vi "UHR-Fleezers Control (host) - Avogadro v3.vi"() -> ()   [LabVIEW 2014] (continued)
  n68 = Bundle("New Image"=w50, "New Image"=w49, "New Image"=w32, "New Image"=w48, "New Image"=w47) -> (w46:T42)  [unwired: 1 in]
  n69 = call-poly "VISA Configure Serial Port"("VISA resource name"=refnum<visa-resource-name> "COM5", "timeout (10sec)"=u32 1000, "baud rate (9600)"=u32 19200) -> ("VISA resource name out"=w3:refnum<visa-resource-name>, "error out"=w6:errorcluster)  [unwired: 4 in, 7 out]
  "Stage Control Serial Error" <- w6
  n70 = node-c288() -> (w53:T43)  [unwired: 4 in]
  n71 = timed-loop "Run Scripts, including: stage motion" {
    tunnel: w6 -> [w231]
    tunnel: w3 -> [w232]
    tunnel: [w232] -> w55
    tunnel: [w231] -> w54
    timing: w53 -> [_]
    timing-out: [_] -> w52
    tunnel: w44 -> [w230]
    tunnel: w45 -> [w229]
    tunnel: w40 -> [w226]
    tunnel: w39 -> [w225]
    tunnel: w38 -> [w227]
    tunnel: w37 -> [w228]
    tunnel: w29 -> [w224]
    tunnel: w26 -> [w223]
    tunnel: w14 -> [w222]
    tunnel: w13 -> [w221]
    stop <- w233 stop-if-true
    n72 = node-c288() -> ()  [unwired: 1 in, 1 out]
    n73 = event shown="[13] \"Cal/Data Acq. Spot\": Value Change" {
      selector: _ -> [_ _ _ _ _ _ _ _ _ _ _ _ _ _ _ _ _ _ _ _ _ _ _ _ _ _ _]
      dyn-events: _ -> [_ _ _ _ _ _ _ _ _ _ _ _ _ _ _ _ _ _ _ _ _ _ _ _ _ _ _]
      timeout: _ -> [_ _ _ _ _ _ _ _ _ _ _ _ _ _ _ _ _ _ _ _ _ _ _ _ _ _ _]
      tunnel: ["Set Position" _ "Move to Position" _ _ _ _ _ _ "Read Harvard" _ _ _ _ _ _ _ _ "Force FB Data\nScript" _ _ "Take Stepping Data" _ "Take Detection Laser\nImage" _ _ _] -> _
      tunnel: [_ _ _ _ _ _ _ _ _ _ _ _ _ _ _ _ _ _ _ _ _ _ _ _ _ w1240 _] -> w233
      tunnel: w231 -> [w252 w260 w271 w284 w314 _ _ _ _ _ w451 w485 w511 w544 w653 w682 w814 w842 w873 _ _ _ _ _ _ _ _]
      tunnel: w232 -> [w253 w261 w272 w285 w315 _ _ _ _ _ w452 w486 w512 w545 w654 w683 w815 w843 w874 _ _ _ _ _ _ _ _]
      tunnel: w230 -> [_ _ _ _ _ _ _ _ _ w436 _ _ _ _ _ _ _ _ _ _ _ _ _ _ _ _ _]
      tunnel: w229 -> [_ _ _ _ _ _ _ _ _ w435 _ _ _ _ _ _ _ _ _ _ _ _ _ _ _ _ _]
      tunnel: w228 -> [_ _ _ _ _ _ _ _ _ _ _ _ _ _ _ _ _ _ _ _ _ _ _ _ _ _ _]
      tunnel: w227 -> [_ _ _ _ _ _ _ _ _ _ _ _ _ _ _ _ _ _ _ _ _ _ _ _ _ _ _]
      tunnel: w226 -> [_ _ _ _ _ _ _ _ _ _ _ _ _ _ _ _ _ _ _ _ _ _ _ _ _ _ _]
      tunnel: w225 -> [_ _ _ _ _ _ _ _ _ _ _ _ _ _ _ _ _ _ _ _ _ _ _ _ _ _ _]
      tunnel: w224 -> [_ _ _ _ _ w342 w349 w377 w396 _ _ _ _ _ _ _ _ _ _ _ _ _ _ _ _ w1239 _]
      tunnel: w223 -> [_ _ _ _ _ _ _ _ _ _ _ _ _ w537 _ _ _ _ _ _ _ _ _ _ w1106 _ _]
      tunnel: w222 -> [_ _ _ _ _ _ _ _ _ _ _ _ _ _ _ _ _ _ _ _ _ _ _ _ _ _ w1250]
      tunnel: w221 -> [_ _ _ _ _ _ _ _ _ _ _ _ _ _ _ _ _ _ _ _ _ _ _ _ _ _ w1245]
      event "Set Position", "Set Position 2", "Set Position 3", "Set Position 4", "Set Position 5", "Set Position 1", "Set Position 6": Value Change {
        n74 = event-data() -> ()  [unwired: 1 in, 5 out]
        n75 = Build Array("Set Position 1", "Set Position 2", "Set Position 3", "Set Position 4", "Set Position 5", "Set Position 6") -> (w251:bool[])
        n76 = Boolean Array To Number(Boolean array=w251) -> (number=w250:u32)
        n77 = Logarithm Base 2(1:w250) -> (0:w242:dbl)
        n78 = call "Read Stage Position.vi"("error in"=w252, "VISA resource name in"=w253) -> ("Current Position"=w257:cluster{dbl, dbl, dbl}, "error out"=w256:errorcluster)  [unwired: 2 out]
        n79 = Decrement(x="Position") -> (x-1=w240:dbl)
        n80 = Greater Or Equal?(x=w242, y=0.0) -> (x >= y?=w243:bool)
        n81 = Cluster To Array(cluster=w257) -> (array=w254:dbl[])
        n82 = Select(t=w242, s=w243, f=w240) -> (s? t:f=w239:dbl)
        n83 = local write "Stage Control Serial Error"(w256) -> ()
        n84 = Increment(x=w239) -> (x+1=w238:dbl)
        n85 = Build Array (concatenate)(w238, w254) -> (w237:dbl[])
        n86 = Replace Array Subset(array="Saved Stage Positions", new element=w237, index (row)=w239) -> (w255:dbl[][])  [unwired: 1 in]
        n87 = local write "Saved Stage Positions"(w255) -> ()
      }
      event Menu Selection (User) {
        n88 = event-data() -> ("ItemTag"=w262:string)  [unwired: 1 in, 6 out]
        n89 = case shown="\"Z\"" w262 {
          tunnel: w261 -> [_ w264 w269 _]
          tunnel: w260 -> [_ w263 w267 _]
          frame "False", Default {
          }
          frame "XY" {
            n90 = call "start_stage_trackball.vi"("Enum"=T46."Trackball XY", "error in (no error)"=w263, "Stage Controller port"=w264) -> ("error out"=w266:errorcluster)  [unwired: 1 out]
            n91 = property on="Stage Control Serial Error" class="Clust (strict)"("Val(Sgnl)"=w266) -> ()  [unwired: 2 in, 2 out]
          }
          frame "Z" {
            n92 = call "start_stage_trackball.vi"("Enum"=T46."Trackball Z", "error in (no error)"=w267, "Stage Controller port"=w269) -> ("error out"=w268:errorcluster)  [unwired: 1 out]
            n93 = property on="Stage Control Serial Error" class="Clust (strict)"("Val(Sgnl)"=w268) -> ()  [unwired: 2 in, 2 out]
          }
          frame "True" {
          }
        }
      }
      event "Move to Position": Value Change {
        n94 = event-data() -> ()  [unwired: 1 in, 5 out]
        n95 = flat-sequence {
          tunnel: w272 -> [w276]
          tunnel: w271 -> [w275]
          frame #0 {
            n96 = local read "Saved Stage Positions"() -> (w278:dbl[][])
            n97 = local read "Position"() -> (w277:dbl)
            n98 = local write "Stage Moving"(TRUE ("Stage Moving")) -> ()
            n99 = call "move to saved stage position.vi"("error in"=w275, "Stage VISA resource name in"=w276, "Position"=w277, "Saved Stage Positions"=w278) -> ("error out"=w274:errorcluster)  [unwired: 1 out]
            n100 = local write "Stage Control Serial Error"(w274) -> ()
          }
          frame #1 {
            n101 = call <vilib>:"Beep.vi"() -> ()  [unwired: 3 in, 9 out]
            n102 = local write "Stage Moving"(FALSE ("Stage Moving")) -> ()
          }
        }
      }
      event "Move Cap. 1 (DNA Bottom)": Value Change {
        n103 = event-data() -> ()  [unwired: 1 in, 5 out]
        n104 = local write "Move Cap. 1 (DNA Bottom)"(FALSE ("Move Cap. 1 (DNA Right)")) -> ()
        n105 = flat-sequence {
          tunnel: w284 -> [w287]
          tunnel: w285 -> [w288]
          tunnel: [w288] -> w282
          tunnel: [w287] -> w281
          tunnel: w282 -> [w290]
          tunnel: w281 -> [w289]
          frame #0 {
            n106 = property on="Sample Channel\nFlow" class="Bool (strict)"("Val(Sgnl)"="Cap 1 Samp Flow ON") -> ()  [unwired: 2 in, 2 out]
          }
          frame #1 {
            n107 = local read "Saved Stage Positions"() -> (w300:dbl[][])
            n108 = local write "Stage Moving"(TRUE ("Stage Moving")) -> ()
            n109 = Array Subset(array=w300, index (row)=0 ("index"), length (row)=1 ("length"), index (col)=1 ("index"), length (col)=3 ("length")) -> (w297:dbl[][])
            n110 = Reshape Array(w297, 3 ("dimension size")) -> (w295:dbl[])
            n111 = Array To Cluster(array=w295) -> (cluster=w294:cluster{"[0]":dbl, "[1]":dbl, "[2]":dbl})
            n112 = call "Set Stage Position.vi"("Position"=w294, "error in"=w289, "VISA resource name in"=w290) -> ("error out"=w293:errorcluster)  [unwired: 2 out]
            n113 = local write "Stage Control Serial Error"(w293) -> ()
          }
          frame #2 {
            n114 = local write "Stage Moving"(FALSE ("Stage Moving")) -> ()
            n115 = case shown="True" "Cap 1 Flow ON" {
              frame False {
              }
              frame True {
                n116 = property on="Inject Pump 1" class="Bool (strict)"("Val(Sgnl)"=TRUE ("Value (Signaling)")) -> ()  [unwired: 2 in, 2 out]
              }
            }
            n117 = call <vilib>:"Beep.vi"() -> ()  [unwired: 3 in, 9 out]
          }
          frame #3 {
            n118 = property on="Sample Channel\nFlow" class="Bool (strict)"("Val(Sgnl)"=FALSE ("Value (Signaling)")) -> ()  [unwired: 2 in, 2 out]
            n119 = local read "Cap. 2 BD T1?\n(ADig T1, DNA T2)"() -> (w307:bool)
            n120 = case shown="True" w307 {
              tunnel: "Cap 1 T ON" -> [w309 w310]
              frame False {
                n121 = property on="Trap 1 (ON/OFF)" class="Bool (strict)"("Val(Sgnl)"=w309) -> ()  [unwired: 2 in, 2 out]
              }
              frame True {
                n122 = property on="Trap 2 (ON/OFF)" class="Bool (strict)"("Val(Sgnl)"=w310) -> ()  [unwired: 2 in, 2 out]
              }
            }
            n123 = property on="Get bead 2" class="Bool (strict)"("Key Focus"=TRUE) -> ()  [unwired: 2 in, 2 out]
          }
        }
      }
      event "Move Cap. 2 (ADig Top)": Value Change {
        n124 = event-data() -> ()  [unwired: 1 in, 5 out]
        n125 = local write "Move Cap. 2 (ADig Top)"(FALSE ("Move Cap. 2 (ADig Left)")) -> ()
        n126 = flat-sequence {
          tunnel: w314 -> [w317]
          tunnel: w315 -> [w318]
          tunnel: [w318] -> w312
          tunnel: [w317] -> w311
          tunnel: w312 -> [w321]
          tunnel: w311 -> [w320]
          frame #0 {
            n127 = property on="Sample Channel\nFlow" class="Bool (strict)"("Val(Sgnl)"="Cap 2 Samp Flow ON") -> ()  [unwired: 2 in, 2 out]
          }
          frame #1 {
            w319 = FALSE ("Value (Signaling)")
            n128 = local read "Saved Stage Positions"() -> (w331:dbl[][])
            n129 = local write "Stage Moving"(TRUE ("Stage Moving")) -> ()
            n130 = Array Subset(array=w331, index (row)=1 ("index"), length (row)=1 ("length"), index (col)=1 ("index"), length (col)=3 ("length")) -> (w328:dbl[][])
            n131 = Reshape Array(w328, 3 ("dimension size")) -> (w326:dbl[])
            n132 = property on="Trap 1 (ON/OFF)" class="Bool (strict)"("Val(Sgnl)"=w319) -> ()  [unwired: 2 in, 2 out]
            n133 = property on="Trap 1 (ON/OFF)" class="Bool (strict)"("Val(Sgnl)"=w319) -> ()  [unwired: 2 in, 2 out]
            n134 = Array To Cluster(array=w326) -> (cluster=w325:cluster{"[0]":dbl, "[1]":dbl, "[2]":dbl})
            n135 = call "Set Stage Position.vi"("Position"=w325, "error in"=w320, "VISA resource name in"=w321) -> ("error out"=w324:errorcluster)  [unwired: 2 out]
            n136 = local write "Stage Control Serial Error"(w324) -> ()
          }
          frame #2 {
            n137 = local write "Stage Moving"(FALSE ("Stage Moving")) -> ()
            n138 = call <vilib>:"Beep.vi"() -> ()  [unwired: 3 in, 9 out]
            n139 = case shown="True" "Cap 2 Flow ON" {
              frame False {
              }
              frame True {
                n140 = property on="Inject Pump 3" class="Bool (strict)"("Val(Sgnl)"=TRUE ("Value (Signaling)")) -> ()  [unwired: 2 in, 2 out]
              }
            }
          }
          frame #3 {
            n141 = property on="Sample Channel\nFlow" class="Bool (strict)"("Val(Sgnl)"=FALSE ("Value (Signaling)")) -> ()  [unwired: 2 in, 2 out]
            n142 = case shown="False" "Cap. 2 BD T1?\n(ADig T1, DNA T2)" {
              tunnel: "Cap 2 T ON" -> [w340 w341]
              frame False {
                n143 = property on="Trap 2 (ON/OFF)" class="Bool (strict)"("Val(Sgnl)"=w340) -> ()  [unwired: 2 in, 2 out]
              }
              frame True {
                n144 = property on="Trap 1 (ON/OFF)" class="Bool (strict)"("Val(Sgnl)"=w341) -> ()  [unwired: 2 in, 2 out]
              }
            }
            n145 = property on="Get bead 3" class="Bool (strict)"("Key Focus"=TRUE) -> ()  [unwired: 2 in, 2 out]
          }
        }
      }
      event "Send string\nto Blue Laser": Value Change {
        n146 = event-data() -> ()  [unwired: 1 in, 5 out]
        n147 = flat-sequence {
          tunnel: w342 -> [w343]
          frame #0 {
            n148 = call "serial write macro.vi"("String"="command string", "Delay (ms)"="Delay (ms)", "VISA resource name"=w343) -> ("read buffer"=→"read blue buffer":string, "error out"=→"Blue Error Out":errorcluster)  [unwired: 1 out]
            "command string sent" <- "command string"
          }
          frame #1 {
            n149 = local write "Send string\nto Blue Laser"(FALSE ("Send string")) -> ()
          }
        }
      }
      event "Get Blue Laser State": Value Change {
        n150 = event-data() -> ()  [unwired: 1 in, 5 out]
        n151 = local read "Delay (ms)"() -> (w350:i32)
        n152 = flat-sequence {
          tunnel: w350 -> [w358]
          tunnel: w349 -> [w361]
          tunnel: [w359] -> w354
          tunnel: [w358] -> w353
          tunnel: [w368] -> w352
          tunnel: [w365] -> w351
          tunnel: w354 -> [w366]
          tunnel: w353 -> [w365]
          tunnel: w352 -> [w374]
          tunnel: w351 -> [w372]
          frame #0 {
            w356 = "l?"
            n153 = local write "command string sent"(w356) -> ()
            n154 = call "serial write macro.vi"("String"=w356, "Delay (ms)"=w358, "VISA resource name"=w361) -> ("read buffer"=w357:string, "VISA resource name out"=w359:refnum<visa-resource-name>)  [unwired: 1 out]
            n155 = Decimal String To Number(string=w357) -> (number=w360:i32)  [unwired: 2 in, 1 out]
            n156 = Not Equal To 0?(x=w360) -> (x != 0?=→"Laser On":bool)
            n157 = local write "read blue buffer"(w357) -> ()
          }
          frame #1 {
            w363 = "games?" ("String")
            n158 = local write "command string sent"(w363) -> ()
            n159 = call "serial write macro.vi"("String"=w363, "Delay (ms)"=w365, "VISA resource name"=w366) -> ("read buffer"=w364:string, "VISA resource name out"=w368:refnum<visa-resource-name>)  [unwired: 1 out]
            n160 = Decimal String To Number(string=w364) -> (number=w367:i32)  [unwired: 2 in, 1 out]
            n161 = local write "read blue buffer"(w364) -> ()
            n162 = Not Equal To 0?(x=w367) -> (x != 0?=→"Analog Modulation":bool)
          }
          frame #2 {
            w370 = "gdmes?" ("String")
            n163 = local write "command string sent"(w370) -> ()
            n164 = call "serial write macro.vi"("String"=w370, "Delay (ms)"=w372, "VISA resource name"=w374) -> ("read buffer"=w371:string)  [unwired: 2 out]
            n165 = Decimal String To Number(string=w371) -> (number=w373:i32)  [unwired: 2 in, 1 out]
            n166 = Not Equal To 0?(x=w373) -> (x != 0?=→"Digital Modulation":bool)
            n167 = local write "read blue buffer"(w371) -> ()
          }
          frame #3 {
            n168 = local write "Get Blue Laser State"(FALSE) -> ()
          }
        }
      }
      event "Blue Laser Power (mW)\n(Constant Power Mode)", "Blue Laser Modulation\nPower (mW)": Value Change {
        n169 = event-data() -> ()  [unwired: 1 in, 5 out]
        n170 = flat-sequence {
          tunnel: w377 -> [w383]
          tunnel: [w381] -> w376
          tunnel: w376 -> [w390]
          frame #0 {
            n171 = local read "Delay (ms)"() -> (w382:i32)
            n172 = Concatenate Strings("slmp " ("string"), "Blue Laser Modulation\nPower (mW)") -> (w378:string)
            n173 = call "serial write macro.vi"("String"=w378, "Delay (ms)"=w382, "VISA resource name"=w383) -> ("read buffer"=w379:string, "error out"=w380:errorcluster, "VISA resource name out"=w381:refnum<visa-resource-name>)
            n174 = local write "command string sent"(w378) -> ()
            n175 = local write "read blue buffer"(w379) -> ()
            n176 = local write "Blue Error Out"(w380) -> ()
          }
          frame #1 {
            n177 = local read "Delay (ms)"() -> (w389:i32)
            n178 = Concatenate Strings("p " ("string"), "Blue Laser Power (mW)\n(Constant Power Mode)") -> (w386:string)
            n179 = call "serial write macro.vi"("String"=w386, "Delay (ms)"=w389, "VISA resource name"=w390) -> ("read buffer"=w387:string, "error out"=w388:errorcluster)  [unwired: 1 out]
            n180 = local write "command string sent"(w386) -> ()
            n181 = local write "read blue buffer"(w387) -> ()
            n182 = local write "Blue Error Out"(w388) -> ()
          }
        }
      }
      event "Laser interlacing mode", "Blue Laser Modulation Mode", "Blue Laser ON": Value Change {
        n183 = event-data() -> ()  [unwired: 1 in, 5 out]
        n184 = flat-sequence {
          tunnel: w396 -> [w401]
          tunnel: [w400] -> w393
          tunnel: [w406] -> w395
          tunnel: w393 -> [w409]
          tunnel: w395 -> [w421]
          tunnel: [w415] -> w394
          tunnel: w394 -> [w428]
          frame #0 {
            n185 = local read "Blue Laser ON"() -> (w398:bool)
            n186 = local read "Delay (ms)"() -> (w399:i32)
            n187 = case shown="False" w398 {
              tunnel: ["l0" "l1"] -> w397
              frame False {
              }
              frame True {
              }
            }
            n188 = call "serial write macro.vi"("String"=w397, "Delay (ms)"=w399, "VISA resource name"=w401) -> ("error out"=w402:errorcluster, "VISA resource name out"=w400:refnum<visa-resource-name>)  [unwired: 1 out]
            n189 = local write "Blue Error Out"(w402) -> ()
          }
          frame #1 {
            n190 = local read "Laser interlacing mode"() -> (w411:enum32{"Laser ON", "Laser OFF", "Interlace"})
            n191 = case shown="\"Laser ON\"" w411 {
              tunnel: ["cp" "em" "l0"] -> w405
              frame "Laser ON" {
              }
              frame "Interlace" {
              }
              frame "Laser OFF", Default {
              }
            }
            n192 = local read "Delay (ms)"() -> (w410:i32)
            n193 = call "serial write macro.vi"("String"=w405, "Delay (ms)"=w410, "VISA resource name"=w409) -> ("read buffer"=w407:string, "error out"=w408:errorcluster, "VISA resource name out"=w406:refnum<visa-resource-name>)
            n194 = local write "command string sent"(w405) -> ()
            n195 = local write "read blue buffer"(w407) -> ()
            n196 = local write "Blue Error Out"(w408) -> ()
          }
          frame #2 {
            n197 = case shown="\"Analog Modulation\"" "Blue Laser Modulation Mode" {
              tunnel: ["sdmes 0" "sdmes 1" "sdmes 1"] -> w416
              frame "Analog Modulation" {
              }
              frame "Digital + Analog Modulation" {
              }
              frame "Digital Modulation", Default {
              }
            }
            n198 = local read "Delay (ms)"() -> (w419:i32)
            n199 = call "serial write macro.vi"("String"=w416, "Delay (ms)"=w419, "VISA resource name"=w421) -> ("read buffer"=w417:string, "error out"=w418:errorcluster, "VISA resource name out"=w415:refnum<visa-resource-name>)
            n200 = local write "command string sent"(w416) -> ()
            n201 = local write "read blue buffer"(w417) -> ()
            n202 = local write "Blue Error Out"(w418) -> ()
          }
          frame #3 {
            n203 = local read "Blue Laser Modulation Mode"() -> (w430:string)
            n204 = case shown="\"Digital Modulation\", Default" w430 {
              tunnel: ["sames 1" "sames 1" "sames 0"] -> w426
              frame "Analog Modulation" {
              }
              frame "Digital + Analog Modulation" {
              }
              frame "Digital Modulation", Default {
              }
            }
            n205 = local read "Delay (ms)"() -> (w429:i32)
            n206 = local write "command string sent"(w426) -> ()
            n207 = call "serial write macro.vi"("String"=w426, "Delay (ms)"=w429, "VISA resource name"=w428) -> ("read buffer"=w427:string, "error out"=w425:errorcluster)  [unwired: 1 out]
            n208 = local write "read blue buffer"(w427) -> ()
            n209 = local write "Blue Error Out"(w425) -> ()
          }
        }
      }
      event "Read Harvard": Value Change {
        n210 = event-data() -> ()  [unwired: 1 in, 5 out]
        n211 = Concatenate Strings("write buffer", "\r") -> (w438:string)
        n212 = VISA Write(VISA resource name=w436, write buffer=w438, error in (no error)=w435) -> (VISA resource name out=w447:refnum<visa-resource-name>, error out=w446:errorcluster)  [unwired: 1 out]
        n213 = stacked-sequence {
          tunnel: [w450] -> w445
          tunnel: w447 -> [w450]
          tunnel: w446 -> [w449]
          tunnel: [w449] -> w440
          frame #0 {
            n214 = Wait (ms)(milliseconds to wait=50) -> ()  [unwired: 1 out]
          }
        }
        n215 = property class="Instr"(reference=w445, error in=w440) -> (reference out=w444:refnum<visa-resource-name>, error out=w442:errorcluster, "Serial Settings:Number of Bytes at Serial Port"=w443:u32)
        "Serial Settings:Number of Bytes at Serial Port" <- w443
        n216 = VISA Read(VISA resource name=w444, byte count=w443, error in (no error)=w442) -> (read buffer=w441:string)  [unwired: 3 out]
        "read buffer" <- w441
        n217 = Fract/Exp String To Number(string=w441) -> ()  [unwired: 5 out]
      }
      event "+z", "-z": Value Change {
        n218 = event-data() -> ()  [unwired: 1 in, 5 out]
        n219 = flat-sequence {
          tunnel: w451 -> [w473]
          tunnel: w452 -> [w453]
          frame #0 {
            n220 = call "Read Stage Position.vi"("error in"=w473, "VISA resource name in"=w453) -> ("Current Position"=w458:cluster{dbl, dbl, dbl}, "error out"=w471:errorcluster, "VISA resource name out"=w472:refnum<visa-resource-name>)  [unwired: 1 out]
            n221 = local read "Saved Stage Positions"() -> (w482:dbl[][])
            n222 = Divide(x="z nudge increment (um)", y=1000.0) -> (x/y=w470:dbl)
            n223 = Boolean To (0,1)(Boolean="+z") -> (0, 1=w462:i16)
            n224 = Boolean To (0,1)(Boolean="-z") -> (0, 1=w463:i16)
            n225 = Array Subset(array=w482, index (row)=1 ("index"), length (row)=1 ("length"), index (col)=1 ("index"), length (col)=3 ("length")) -> (w479:dbl[][])
            n226 = Multiply(x=w462, y=w470) -> (x*y=w466:dbl)
            n227 = Multiply(x=w463, y=w470) -> (x*y=w464:dbl)
            n228 = Unbundle(w458) -> (w456:dbl, w455:dbl, w459:dbl)
            n229 = Negate(x=w464) -> (-x=w465:dbl)
            n230 = Reshape Array(w479, 3 ("dimension size")) -> (w477:dbl[])
            n231 = Add(x=w466, y=w465) -> (x+y=w467:dbl)
            n232 = Array To Cluster(array=w477) -> ()  [unwired: 1 out]
            n233 = Add(x=w467, y=w459) -> (x+y=w457:dbl)
            n234 = Bundle(cluster=w458, w456, w455, w457) -> (w454:cluster{dbl, dbl, dbl})
            n235 = call "Set Stage Position.vi"("Position"=w454, "error in"=w471, "VISA resource name in"=w472) -> ("error out"=w476:errorcluster)  [unwired: 2 out]
            n236 = local write "Stage Moving"(TRUE ("Stage Moving")) -> ()
            n237 = local write "Stage Control Serial Error"(w476) -> ()
          }
          frame #1 {
            n238 = local write "Stage Moving"(FALSE ("Stage Moving")) -> ()
          }
        }
      }
      event "-y", "+y": Value Change {
        n239 = event-data() -> ()  [unwired: 1 in, 5 out]
        n240 = flat-sequence {
          tunnel: w485 -> [w509]
          tunnel: w486 -> [w492]
          frame #0 {
            n241 = call "Read Stage Position.vi"("error in"=w509, "VISA resource name in"=w492) -> ("Current Position"=w495:cluster{dbl, dbl, dbl}, "error out"=w507:errorcluster, "VISA resource name out"=w508:refnum<visa-resource-name>)  [unwired: 1 out]
            n242 = Divide(x="y nudge increment (um", y=1000.0) -> (x/y=w506:dbl)
            n243 = Boolean To (0,1)(Boolean="+y") -> (0, 1=w498:i16)
            n244 = Boolean To (0,1)(Boolean="-y") -> (0, 1=w499:i16)
            n245 = Multiply(x=w498, y=w506) -> (x*y=w502:dbl)
            n246 = Multiply(x=w499, y=w506) -> (x*y=w500:dbl)
            n247 = Unbundle(w495) -> (w494:dbl, w489:dbl, w491:dbl)
            n248 = Negate(x=w500) -> (-x=w501:dbl)
            n249 = Add(x=w502, y=w501) -> (x+y=w503:dbl)
            n250 = Add(x=w503, y=w489) -> (x+y=w490:dbl)
            n251 = Bundle(cluster=w495, w494, w490, w491) -> (w493:cluster{dbl, dbl, dbl})
            n252 = call "Set Stage Position.vi"("Position"=w493, "error in"=w507, "VISA resource name in"=w508) -> ("error out"=w488:errorcluster)  [unwired: 2 out]
            n253 = local write "Stage Control Serial Error"(w488) -> ()
            n254 = local write "Stage Moving"(TRUE ("Stage Moving")) -> ()
          }
          frame #1 {
            n255 = local write "Stage Moving"(FALSE ("Stage Moving")) -> ()
          }
        }
      }
      event "-x", "+x": Value Change {
        n256 = event-data() -> ()  [unwired: 1 in, 5 out]
        n257 = flat-sequence {
          tunnel: w511 -> [w535]
          tunnel: w512 -> [w519]
          frame #0 {
            n258 = call "Read Stage Position.vi"("error in"=w535, "VISA resource name in"=w519) -> ("Current Position"=w521:cluster{dbl, dbl, dbl}, "error out"=w533:errorcluster, "VISA resource name out"=w534:refnum<visa-resource-name>)  [unwired: 1 out]
            n259 = Divide(x="x nudge increment (um)", y=1000.0) -> (x/y=w532:dbl)
            n260 = Boolean To (0,1)(Boolean="+x") -> (0, 1=w524:i16)
            n261 = Boolean To (0,1)(Boolean="-x") -> (0, 1=w525:i16)
            n262 = Multiply(x=w524, y=w532) -> (x*y=w528:dbl)
            n263 = Multiply(x=w525, y=w532) -> (x*y=w526:dbl)
            n264 = Unbundle(w521) -> (w513:dbl, w515:dbl, w518:dbl)
            n265 = Negate(x=w526) -> (-x=w527:dbl)
            n266 = Add(x=w528, y=w527) -> (x+y=w529:dbl)
            n267 = Add(x=w529, y=w513) -> (x+y=w514:dbl)
            n268 = Bundle(cluster=w521, w514, w515, w518) -> (w520:cluster{dbl, dbl, dbl})
            n269 = call "Set Stage Position.vi"("Position"=w520, "error in"=w533, "VISA resource name in"=w534) -> ("error out"=w516:errorcluster)  [unwired: 2 out]
            n270 = local write "Stage Control Serial Error"(w516) -> ()
            n271 = local write "Stage Moving"(TRUE ("Stage Moving")) -> ()
          }
          frame #1 {
            n272 = local write "Stage Moving"(FALSE ("Stage Moving")) -> ()
          }
        }
      }
      event "Cal/Data Acq. Spot": Value Change {
        # "03-01-2018 Changed by RG to incorporate offset measurements at multiple \npositions of the piezo mirror"
        # "Disabled by Ronen - we have our own way of controlling the location of calibration."
        n273 = event-data() -> ()  [unwired: 1 in, 5 out]
        n274 = flat-sequence {
          tunnel: w544 -> [w548]
          tunnel: w545 -> [w549]
          tunnel: [w549] -> w541
          tunnel: [w548] -> w540
          tunnel: w541 -> [w552]
          tunnel: w540 -> [w551]
          tunnel: ["Cal @ (MHz)"] -> w538
          tunnel: [w560] -> w542
          tunnel: w538 -> [w560]
          tunnel: w542 -> [w574]
          tunnel: ["W/ Offset 1"] -> w539
          tunnel: w537 -> [w572]
          tunnel: w542 -> [w614]
          tunnel: w539 -> [w612]
          frame #0 {
            n275 = property on="Sample Channel\nFlow" class="Bool (strict)"("Val(Sgnl)"="Daq spot flow on") -> ()  [unwired: 2 in, 2 out]
            n276 = Wait (ms)(milliseconds to wait=u32 250) -> ()  [unwired: 1 out]
          }
          frame #1 {
            n277 = disable-structure shown="Disabled" {
              disable-tunnel: w552 -> [w557 _]
              disable-tunnel: w551 -> [w556 _]
              frame Disabled {
                n278 = local read "Saved Stage Positions"() -> (w554:dbl[][])
                n279 = call "move to saved stage position.vi"("error in"=w556, "Stage VISA resource name in"=w557, "Position"="Cal Stage Position", "Saved Stage Positions"=w554) -> ("error out"=w555:errorcluster)  [unwired: 1 out]
                n280 = local write "Stage Control Serial Error"(w555) -> ()
              }
              frame Enabled {
              }
            }
            n281 = property on="Trap Delta (MHz)" class="DigNum (strict)"("Val(Sgnl)"="Cal @ (MHz)") -> ()  [unwired: 2 in, 2 out]
            n282 = local write "Stage Moving"(TRUE ("Stage Moving")) -> ()
          }
          frame #2 {
            n283 = local write "Stage Moving"(FALSE ("Stage Moving")) -> ()
            n284 = property on="Sample Channel\nFlow" class="Bool (strict)"("Val(Sgnl)"="Flow ON during cal?") -> ()  [unwired: 2 in, 2 out]
            n285 = call <vilib>:"Beep.vi"() -> ()  [unwired: 3 in, 9 out]
          }
          frame #3 {
            n286 = Wait (ms)(milliseconds to wait=u32 1000) -> ()  [unwired: 1 out]
          }
          frame #4 {
            n287 = case shown="False" "Active cal after cal?" {
              frame False {
              }
              frame True {
                n288 = local write "Active Cal"(TRUE ("Active Cal")) -> ()
                n289 = Wait (ms)(milliseconds to wait=u32 8000) -> ()  [unwired: 1 out]
              }
            }
          }
          frame #5 {
            n290 = property on="Save Calibration" class="Bool (strict)"("Val(Sgnl)"=TRUE ("Value (Signaling)")) -> ()  [unwired: 2 in, 2 out]
          }
          frame #6 {
            n291 = Wait (ms)(milliseconds to wait=u32 2000) -> ()  [unwired: 1 out]
          }
          frame #7 {
            # "Check to see if \nsaving done"
            n292 = while {
              stop <- w568 stop-if-true
              n293 = local read "Saving..."() -> (w569:bool)
              n294 = Wait (ms)(milliseconds to wait=u32 100) -> ()  [unwired: 1 out]
              n295 = Not(x=w569) -> (.not. x?=w568:bool)
            }
          }
          frame #8 {
            n296 = case shown="True" "W/ Offset 1" {
              tunnel: w574 -> [_ w577]
              tunnel: w572 -> [_ w576]
              tunnel: "Multiple-MCL offset?" -> [_ w575]
              frame False {
              }
              frame True {
                n297 = stacked-sequence {
                  tunnel: w577 -> [_ _ _ _ _ _ _ _ _ w610 _]
                  tunnel: w576 -> [_ _ _ _ w588 _ _ _ _ w608 _]
                  tunnel: w575 -> [_ _ _ _ w587 _ _ _ _ _ _]
                  frame #0 {
                    n298 = property on="Trap Delta (MHz)" class="DigNum (strict)"("Val(Sgnl)"="Offset 1 Start (MHz)") -> ()  [unwired: 2 in, 2 out]
                    n299 = Replace Array Subset(array=u32[] [0] ("Index Values"), new element="Offset 1 Set", index=0) -> (w579:u32[])
                    n300 = property on="Saved AOD Raster Scan Parameter Sets" class="Arr (strict)"("Index Values"=w579) -> ()  [unwired: 2 in, 2 out]
                    n301 = property on="manual raster set" class="Ring (strict)"("Value"="Offset 1 Set") -> ()  [unwired: 2 in, 2 out]
                  }
                  frame #1 {
                    n302 = Wait (ms)(milliseconds to wait=u32 200) -> ()  [unwired: 1 out]
                  }
                  frame #2 {
                    n303 = property on="Load parameters" class="Bool (strict)"("Val(Sgnl)"=TRUE ("Value (Signaling)")) -> ()  [unwired: 2 in, 2 out]
                  }
                  frame #3 {
                    n304 = Wait (ms)(milliseconds to wait=u32 200) -> ()  [unwired: 1 out]
                  }
                  frame #4 {
                    n305 = case shown="True" w587 {
                      tunnel: w588 -> [_ w596]
                      frame False {
                      }
                      frame True {
                        n306 = call "Make Trap3 position array.vi"("MCL offset scanning range (V)"="MCL offset scanning range (V)") -> ("Scan increment"=w593:u64, "Min Y"=w594:u64, "Min X"=w595:u64, "X Data points"=w590:u64, "Y data points"=w589:u64)
                        n307 = Multiply(x=w589, y=w590) -> (x*y=w591:u64)
                        n308 = xnode "Read/Write Control"("FPGA VI Reference In"=w596, "Number of scans"=w591, "Piezo offset Y points"=w589, "Piezo offset X points"=w590, "Piezo offset Xmin"=w595, "Piezo Offset Ymin"=w594, "Piezo Offset Increment"=w593, "Multiple trap 3 position offset  file"=TRUE) -> ()  [unwired: 1 in, 2 out]
                        n309 = property on="Number of F/B Scans (AOD)" class="DigNum (strict)"("Val(Sgnl)"=w591) -> ()  [unwired: 2 in, 2 out]
                      }
                    }
                    n310 = local write "Offset raster?"(TRUE) -> ()
                  }
                  frame #5 {
                    n311 = Wait (ms)(milliseconds to wait=u32 200) -> ()  [unwired: 1 out]
                  }
                  frame #6 {
                    n312 = property on="Trap Raster Scan" class="Bool (strict)"("Val(Sgnl)"=TRUE ("Value (Signaling)")) -> ()  [unwired: 2 in, 2 out]
                  }
                  frame #7 {
                    n313 = Wait (ms)(milliseconds to wait=u32 2000) -> ()  [unwired: 1 out]
                  }
                  frame #8 {
                    n314 = while {
                      stop <- w604 stop-if-true
                      n315 = local read "Raster Scanning..."() -> (w606:bool)
                      n316 = local read "Saving..."() -> (w602:bool)
                      n317 = Wait (ms)(milliseconds to wait=u32 100) -> ()  [unwired: 1 out]
                      n318 = Not(x=w602) -> (.not. x?=w601:bool)
                      n319 = Not(x=w606) -> (.not. x?=w603:bool)
                      n320 = And(x=w603, y=w601) -> (x .and. y?=w604:bool)
                    }
                  }
                  frame #9 {
                    n321 = property on="Trap Delta (MHz)" class="DigNum (strict)"("Val(Sgnl)"=w610) -> ()  [unwired: 2 in, 2 out]
                    n322 = xnode "Read/Write Control"("FPGA VI Reference In"=w608, "Multiple trap 3 position offset  file"=FALSE) -> ()  [unwired: 1 in, 2 out]
                    n323 = local write "Offset raster?"(FALSE) -> ()
                  }
                  frame #10 {
                    n324 = Wait (ms)(milliseconds to wait=u32 2000) -> ()  [unwired: 1 out]
                  }
                }
              }
            }
          }
          frame #9 {
            n325 = local read "Save ave N"() -> (w613:dbl)
            n326 = case shown="True" "W/ Offset 2" {
              tunnel: w614 -> [_ w621]
              tunnel: w613 -> [_ w620]
              tunnel: w612 -> [w616 _]
              frame False {
                n327 = case shown="False" w616 {
                  frame False {
                    n328 = Multiply(x="Cal read wait (s)", y=u32 1000 ("milliseconds to wait")) -> (x*y=w618:u32)
                    n329 = Wait (ms)(milliseconds to wait=w618) -> ()  [unwired: 1 out]
                  }
                  frame True {
                  }
                }
              }
              frame True {
                n330 = stacked-sequence {
                  tunnel: w621 -> [_ _ _ _ _ _ _ _ _ w643 _ _]
                  tunnel: w620 -> [_ _ _ _ _ _ _ _ _ w641 _ _]
                  frame #0 {
                    n331 = property on="Save ave N" class="DigNum (strict)"("Val(Sgnl)"=1.0 ("Value (Signaling)")) -> ()  [unwired: 2 in, 2 out]
                  }
                  frame #1 {
                    n332 = Wait (ms)(milliseconds to wait=u32 500) -> ()  [unwired: 1 out]
                  }
                  frame #2 {
                    n333 = property on="Trap Delta (MHz)" class="DigNum (strict)"("Val(Sgnl)"="Offset 2 Start (MHz)") -> ()  [unwired: 2 in, 2 out]
                    n334 = Replace Array Subset(array=u32[] [0] ("Index Values"), new element="Offset 2 Set", index=0) -> (w626:u32[])
                    n335 = property on="Saved AOD Raster Scan Parameter Sets" class="Arr (strict)"("Index Values"=w626) -> ()  [unwired: 2 in, 2 out]
                  }
                  frame #3 {
                    n336 = Wait (ms)(milliseconds to wait=u32 500) -> ()  [unwired: 1 out]
                  }
                  frame #4 {
                    n337 = property on="Load parameters" class="Bool (strict)"("Val(Sgnl)"=TRUE ("Value (Signaling)")) -> ()  [unwired: 2 in, 2 out]
                    n338 = local write "Offset raster?"(TRUE) -> ()
                  }
                  frame #5 {
                    n339 = Wait (ms)(milliseconds to wait=u32 500) -> ()  [unwired: 1 out]
                  }
                  frame #6 {
                    n340 = property on="Trap Raster Scan" class="Bool (strict)"("Val(Sgnl)"=TRUE ("Value (Signaling)")) -> ()  [unwired: 2 in, 2 out]
                  }
                  frame #7 {
                    n341 = Wait (ms)(milliseconds to wait=u32 2000) -> ()  [unwired: 1 out]
                  }
                  frame #8 {
                    n342 = while {
                      stop <- w636 stop-if-true
                      n343 = local read "Raster Scanning..."() -> (w639:bool)
                      n344 = local read "Saving..."() -> (w637:bool)
                      n345 = Wait (ms)(milliseconds to wait=u32 100) -> ()  [unwired: 1 out]
                      n346 = Not(x=w637) -> (.not. x?=w635:bool)
                      n347 = Not(x=w639) -> (.not. x?=w638:bool)
                      n348 = And(x=w638, y=w635) -> (x .and. y?=w636:bool)
                    }
                  }
                  frame #9 {
                    n349 = property on="Trap Delta (MHz)" class="DigNum (strict)"("Val(Sgnl)"=w643) -> ()  [unwired: 2 in, 2 out]
                    n350 = property on="Saved AOD Raster Scan Parameter Sets" class="Arr (strict)"("Index Values"=u32[] [0]) -> ()  [unwired: 2 in, 2 out]
                    n351 = property on="Save ave N" class="DigNum (strict)"("Val(Sgnl)"=w641) -> ()  [unwired: 2 in, 2 out]
                  }
                  frame #10 {
                    n352 = Wait (ms)(milliseconds to wait=u32 500) -> ()  [unwired: 1 out]
                  }
                  frame #11 {
                    n353 = local write "Offset raster?"(FALSE) -> ()
                    n354 = property on="Load parameters" class="Bool (strict)"("Val(Sgnl)"=TRUE ("Value (Signaling)")) -> ()  [unwired: 2 in, 2 out]
                  }
                }
              }
            }
          }
          frame #10 {
            n355 = property on="Read Cal" class="Bool (strict)"("Val(Sgnl)"=TRUE ("Value (Signaling)")) -> ()  [unwired: 2 in, 2 out]
          }
          frame #11 {
            n356 = Wait (ms)(milliseconds to wait=u32 1000) -> ()  [unwired: 1 out]
          }
          frame #12 {
            n357 = property on="Fish for Tether" class="Bool (strict)"("Val(Sgnl)"="Fish after cal?") -> ()  [unwired: 2 in, 2 out]
          }
        }
        n358 = local write "Cal/Data Acq. Spot"(FALSE ("Cal/Data Acq. Spot")) -> ()
      }
      event "Dump Beads": Value Change {
        n359 = event-data() -> ()  [unwired: 1 in, 5 out]
        n360 = flat-sequence {
          tunnel: ["Dump spot flow on?"] -> w650
          tunnel: [w661] -> w651
          tunnel: w650 -> [w661]
          tunnel: w654 -> [w666]
          tunnel: w653 -> [w665]
          tunnel: [w663] -> w652
          tunnel: w651 -> [w663]
          tunnel: w652 -> [w676]
          frame #0 {
            w655 = FALSE ("Value (Signaling)")
            n361 = local read "Saving..."() -> (w657:bool)
            n362 = local write "Dump Beads"(FALSE ("Dump Beads")) -> ()
            n363 = property on="Inject Pump 3" class="Bool (strict)"("Val(Sgnl)"=w655) -> ()  [unwired: 2 in, 2 out]
            n364 = property on="Inject Pump 1" class="Bool (strict)"("Val(Sgnl)"=w655) -> ()  [unwired: 2 in, 2 out]
            n365 = local write "Stop Saving"(w657) -> ()
          }
          frame #1 {
            w658 = FALSE ("Fl. Triggered...")
            n366 = case shown="True" "Dump spot flow on?" {
              frame False {
              }
              frame True {
                n367 = property on="Sample Channel\nFlow" class="Bool (strict)"("Val(Sgnl)"=TRUE ("Stage Moving")) -> ()  [unwired: 2 in, 2 out]
              }
            }
            n368 = local write "Fl. Triggered..."(w658) -> ()
            n369 = local write "Tether"(w658) -> ()
            n370 = property on="Vortran Laser ON" class="Bool (strict)"("Val(Sgnl)"=w658) -> ()  [unwired: 2 in, 2 out]
            n371 = property on="Trap Pos. FB ON" class="Bool (strict)"("Val(Sgnl)"=w658) -> ()  [unwired: 2 in, 2 out]
            n372 = property on="Trap Trig. Fl." class="Bool (strict)"("Val(Sgnl)"=w658) -> ()  [unwired: 2 in, 2 out]
            n373 = property on="Fl. Triggered..." class="Bool (strict)"("Val(Sgnl)"=w658) -> ()  [unwired: 2 in, 2 out]
            n374 = property on="Dip for Protein" class="Bool (strict)"("Val(Sgnl)"=w658) -> ()  [unwired: 2 in, 2 out]
            n375 = property on="Pause dwell" class="Bool (strict)"("Val(Sgnl)"=w658) -> ()  [unwired: 2 in, 2 out]
          }
          frame #2 {
            n376 = property on="Trap Pos. FB Offset Factor" class="DigNum (strict)"("Val(Sgnl)"=i64 0 ("Value (Signaling)")) -> ()  [unwired: 2 in, 2 out]
          }
          frame #3 {
            n377 = local read "Saved Stage Positions"() -> (w667:dbl[][])
            n378 = local write "Stage Moving"(TRUE ("Stage Moving")) -> ()
            n379 = Array Subset(array=w667, index (row)=3 ("index"), length (row)=1 ("length"), index (col)=1 ("index"), length (col)=3 ("length")) -> (w672:dbl[][])
            n380 = Reshape Array(w672, 3 ("dimension size")) -> (w670:dbl[])
            n381 = Array To Cluster(array=w670) -> (cluster=w669:cluster{"[0]":dbl, "[1]":dbl, "[2]":dbl})
            n382 = call "Set Stage Position.vi"("Position"=w669, "error in"=w665, "VISA resource name in"=w666) -> ()  [unwired: 3 out]
          }
          frame #4 {
            w677 = FALSE ("Value (Signaling)")
            n383 = case shown="True" w676 {
              frame False {
              }
              frame True {
                n384 = property on="Sample Channel\nFlow" class="Bool (strict)"("Val(Sgnl)"=FALSE ("Stage Moving")) -> ()  [unwired: 2 in, 2 out]
              }
            }
            n385 = property on="Trap 1 (ON/OFF)" class="Bool (strict)"("Val(Sgnl)"=w677) -> ()  [unwired: 2 in, 2 out]
            n386 = property on="Trap 2 (ON/OFF)" class="Bool (strict)"("Val(Sgnl)"=w677) -> ()  [unwired: 2 in, 2 out]
            n387 = call <vilib>:"Beep.vi"() -> ()  [unwired: 3 in, 9 out]
          }
          frame #5 {
            n388 = property on="Move Cap. 2 (ADig Top)" class="Bool (strict)"("Val(Sgnl)"=TRUE ("Value (Signaling)")) -> ()  [unwired: 2 in, 2 out]
            n389 = property on="Tab Control" class="TabCtl (strict)"("Val(Sgnl)"=T47."Status" ("Value (Signaling)")) -> ()  [unwired: 2 in, 2 out]
          }
        }
      }
      event "Dip for Protein": Value Change {
        n390 = event-data() -> ()  [unwired: 1 in, 5 out]
        n391 = case shown="True" "Dip for Protein" {
          tunnel: w683 -> [_ w685]
          tunnel: w682 -> [_ w684]
          frame False {
          }
          frame True {
            n392 = while {
              tunnel: w685 -> [w696]
              tunnel: w684 -> [w695]
              i -> [w690]
              stop <- w692 stop-if-true
              n393 = Increment(x=w690) -> (x+1=→"Dip #":i32)
              n394 = flat-sequence {
                tunnel: w695 -> [w707]
                tunnel: w696 -> [w708]
                tunnel: [w708] -> w700
                tunnel: [w707] -> w699
                tunnel: [w701] -> w686
                tunnel: [w713] -> w694
                tunnel: [w714] -> w693
                tunnel: w700 -> [w715]
                tunnel: w699 -> [w716]
                tunnel: [w711] -> w687
                tunnel: w686 -> [w711]
                tunnel: [w724] -> w698
                tunnel: w694 -> [w724]
                tunnel: [w723] -> w697
                tunnel: w693 -> [w723]
                tunnel: [w720] -> w691
                tunnel: [w719] -> w688
                tunnel: w687 -> [w719]
                tunnel: w697 -> [w744]
                tunnel: w698 -> [w745]
                tunnel: w691 -> [w746]
                tunnel: w688 -> [w743]
                tunnel: [w802] -> w692
                frame #0 {
                  n395 = local read "Trap Pos. FB ON"() -> (w701:bool)
                  n396 = Compound Arithmetic op=AND("Flow ON\nduring dip?", "FB OFF when \nflow ON", w701) -> (w702:bool)
                  n397 = case shown="True" "Move trap \nbefore dip move?" {
                    frame False {
                    }
                    frame True {
                      n398 = property on="Trap Delta (MHz)" class="DigNum (strict)"("Val(Sgnl)"="Dipping Delta (MHz)") -> ()  [unwired: 2 in, 2 out]
                    }
                  }
                  n399 = property on="Vortran Laser ON" class="Bool (strict)"("Val(Sgnl)"="Green ON\nbefore dip?") -> ()  [unwired: 2 in, 2 out]
                  n400 = property on="Sample Channel\nFlow" class="Bool (strict)"("Val(Sgnl)"="Flow ON\nduring dip?") -> ()  [unwired: 2 in, 2 out]
                  n401 = case shown="True" w702 {
                    frame False {
                    }
                    frame True {
                      n402 = property on="Trap Pos. FB ON" class="Bool (strict)"("Val(Sgnl)"=FALSE ("Value (Signaling)")) -> ()  [unwired: 2 in, 2 out]
                    }
                  }
                }
                frame #1 {
                  n403 = local read "Saved Stage Positions"() -> (w718:dbl[][])
                  n404 = local write "Cancel dwell"(FALSE ("Cancel dwell")) -> ()
                  n405 = call "move to saved stage position.vi"("error in"=w716, "Stage VISA resource name in"=w715, "Position"="Dip Stage \nPosition", "Saved Stage Positions"=w718) -> ("VISA resource name out"=w713:refnum<visa-resource-name>, "error out"=w714:errorcluster)
                }
                frame #2 {
                  n406 = node-c288() -> (w722:T43)  [unwired: 4 in]
                  n407 = timed-loop {
                    timing: w722 -> [_]
                    timing-out: [_] -> w721
                    tunnel: [w728] -> w720
                    i -> [w725]
                    stop <- w729 stop-if-true
                    n408 = node-c288() -> ()  [unwired: 1 in, 1 out]
                    n409 = Greater Or Equal?(x=w725, y="Dip Duration (s)") -> (x >= y?=w737:bool)
                    n410 = local read "Dip for Protein"() -> (w730:bool)
                    n411 = local read "Dump Beads"() -> (w727:bool)
                    n412 = local read "Cancel dwell"() -> (w736:bool)
                    n413 = local read "Pause dwell"() -> (w733:bool)
                    n414 = Not(x=w730) -> (.not. x?=w735:bool)
                    n415 = Compound Arithmetic op=OR(w736, w737, w735) -> (w734:bool)
                    n416 = Select(t=FALSE, s=w733, f=w734) -> (s? t:f=w731:bool)
                    n417 = Not(x=w727) -> (.not. x?=w726:bool)
                    n418 = node-c288() -> ()  [unwired: 1 in, 1 out]
                    n419 = And(x=w730, y=w726) -> (x .and. y?=w728:bool)
                    n420 = Or(x=w731, y=w727) -> (x .or. y?=w729:bool)
                    "Dip Time (s)" <- w725
                  }
                  n421 = node-c288(w721) -> ()  [unwired: 1 out]
                }
                frame #3 {
                  n422 = case shown="True" w746 {
                    tunnel: w745 -> [_ w751]
                    tunnel: w744 -> [_ w750]
                    tunnel: w743 -> [_ w747]
                    frame False {
                    }
                    frame True {
                      n423 = flat-sequence {
                        tunnel: w750 -> [w755]
                        tunnel: w751 -> [w756]
                        tunnel: [w756] -> w749
                        tunnel: [w755] -> w748
                        tunnel: w747 -> [w752]
                        tunnel: w749 -> [w766]
                        tunnel: w748 -> [w765]
                        tunnel: w747 -> [w774]
                        frame #0 {
                          n424 = local read "Sample Channel\nFlow"() -> (w754:bool)
                          n425 = case shown="True" w754 {
                            tunnel: "Flow ON \nduring return\nfrom dip?" -> [w757 w760]
                            tunnel: w752 -> [_ w759]
                            frame False {
                              n426 = case shown="True" w757 {
                                frame False {
                                }
                                frame True {
                                n427 = property on="Sample Channel\nFlow" class="Bool (strict)"("Val(Sgnl)"=TRUE ("Value (Signaling)")) -> ()  [unwired: 2 in, 2 out]
                                }
                              }
                            }
                            frame True {
                              n428 = case shown="False" w760 {
                                tunnel: w759 -> [w761 _]
                                frame False {
                                n429 = property on="Trap Pos. FB ON" class="Bool (strict)"("Val(Sgnl)"=w761) -> ()  [unwired: 2 in, 2 out]
                                n430 = property on="Sample Channel\nFlow" class="Bool (strict)"("Val(Sgnl)"=FALSE ("Value (Signaling)")) -> ()  [unwired: 2 in, 2 out]
                                }
                                frame True {
                                }
                              }
                            }
                          }
                        }
                        frame #1 {
                          # "For turning on green laser before stage reaches lower spot"
                          n431 = case shown="True" "Green ON\nafter start\nreturn?" {
                            frame False {
                            }
                            frame True {
                              n432 = flat-sequence {
                                frame #0 {
                                n433 = Multiply(x="Green delay after \nstart return (s)", y=1000.0) -> (x*y=w771:dbl)
                                n434 = Wait (ms)(milliseconds to wait=w771) -> ()  [unwired: 1 out]
                                }
                                frame #1 {
                                n435 = property on="Vortran Laser ON" class="Bool (strict)"("Val(Sgnl)"=TRUE ("Value (Signaling)")) -> ()  [unwired: 2 in, 2 out]
                                }
                              }
                            }
                          }
                          n436 = local read "Saved Stage Positions"() -> (w769:dbl[][])
                          n437 = local write "Cancel dwell"(FALSE ("Cancel dwell")) -> ()
                          n438 = call "move to saved stage position.vi"("error in"=w765, "Stage VISA resource name in"=w766, "Position"="Return Stage \nPosition", "Saved Stage Positions"=w769) -> ("error out"=w767:errorcluster)  [unwired: 1 out]
                          n439 = local write "Stage Control Serial Error"(w767) -> ()
                        }
                        frame #2 {
                          n440 = property on="Trap Pos. FB ON" class="Bool (strict)"("Val(Sgnl)"=w774) -> ()  [unwired: 2 in, 2 out]
                          n441 = case shown="True" "Green ON \nafter return?" {
                            frame False {
                            }
                            frame True {
                              n442 = property on="Vortran Laser ON" class="Bool (strict)"("Val(Sgnl)"=TRUE ("Value (Signaling)")) -> ()  [unwired: 2 in, 2 out]
                            }
                          }
                          n443 = case shown="True" "Move trap after return?" {
                            frame False {
                            }
                            frame True {
                              n444 = property on="Trap Delta (MHz)" class="DigNum (strict)"("Val(Sgnl)"="Dip Trap Delta 2 (MHz)") -> ()  [unwired: 2 in, 2 out]
                            }
                          }
                          n445 = case shown="True" "Save data after return?" {
                            frame False {
                            }
                            frame True {
                              n446 = property on="Start Saving" class="Bool (strict)"("Val(Sgnl)"=TRUE ("Value (Signaling)")) -> ()  [unwired: 2 in, 2 out]
                            }
                          }
                          n447 = property on="Sample Channel\nFlow" class="Bool (strict)"("Val(Sgnl)"="Flow ON\nduring daq?") -> ()  [unwired: 2 in, 2 out]
                        }
                        frame #3 {
                          n448 = node-c288() -> (w783:T43)  [unwired: 4 in]
                          n449 = timed-loop {
                            timing: w783 -> [_]
                            timing-out: [_] -> w782
                            i -> [w784]
                            stop <- w786 stop-if-true
                            n450 = node-c288() -> ()  [unwired: 1 in, 1 out]
                            n451 = local read "Dump Beads"() -> (w785:bool)
                            n452 = Greater Or Equal?(x=w784, y="Dwell Duration (s)") -> (x >= y?=w791:bool)
                            n453 = local read "Dip for Protein"() -> (w788:bool)
                            n454 = Not(x=w788) -> (.not. x?=w787:bool)
                            n455 = Compound Arithmetic op=OR(w791, "Cancel dwell", w787) -> (w790:bool)
                            n456 = node-c288() -> ()  [unwired: 1 in, 1 out]
                            n457 = Select(t=FALSE, s="Pause dwell", f=w790) -> (s? t:f=w793:bool)
                            n458 = Or(x=w793, y=w785) -> (x .or. y?=w786:bool)
                            "Dwell Time (s)" <- w784
                          }
                          n459 = node-c288(w782) -> ()  [unwired: 1 out]
                        }
                      }
                    }
                  }
                }
                frame #4 {
                  n460 = local read "Dip for Protein"() -> (w803:bool)
                  n461 = local read "Dump Beads"() -> (w800:bool)
                  n462 = local write "Cancel dwell"(FALSE ("Cancel dwell")) -> ()
                  n463 = Not(x=w803) -> (.not. x?=w804:bool)
                  n464 = Not(x="Cont. Repeat Dipping?") -> (.not. x?=w806:bool)
                  n465 = Compound Arithmetic op=OR(w804, w806, w800) -> (w802:bool)
                }
              }
            }
          }
        }
      }
      event "Profile": Value Change {
        n466 = event-data() -> ()  [unwired: 1 in, 5 out]
        n467 = flat-sequence {
          tunnel: w815 -> [w818]
          tunnel: w814 -> [w826]
          tunnel: [w820] -> w813
          tunnel: [w819] -> w812
          tunnel: [w817] -> w810
          tunnel: [w816] -> w807
          tunnel: w813 -> [w833]
          tunnel: w812 -> [w832]
          tunnel: [w830] -> w811
          tunnel: w810 -> [w831]
          tunnel: [w829] -> w809
          tunnel: [w828] -> w808
          tunnel: w807 -> [w828]
          tunnel: w811 -> [w837]
          tunnel: w809 -> [w836]
          tunnel: w808 -> [w835]
          frame #0 {
            n468 = call "Read Stage Position.vi"("error in"=w826, "VISA resource name in"=w818) -> ("Current Position"=w816:cluster{dbl, dbl, dbl}, "error out"=w819:errorcluster, "VISA resource name out"=w817:refnum<visa-resource-name>)  [unwired: 1 out]
            "Current Position" <- w816
            n469 = local write "Stage Control Serial Error"(w819) -> ()
            n470 = Unbundle(w816) -> (w823:dbl, w825:dbl, w821:dbl)
            n471 = Add(x=w825, y="Y change (mm)") -> (x+y=w822:dbl)
            n472 = Bundle(w823, w822, w821) -> (w820:cluster{dbl, dbl, dbl})  [unwired: 1 in]
          }
          frame #1 {
            # "move to new position and start saving"
            n473 = local write "Stage Moving"(TRUE ("Stage Moving")) -> ()
            n474 = local write "Start Saving"(TRUE ("Start Saving")) -> ()
            n475 = call "Set Stage Position.vi"("Position"=w833, "error in"=w832, "VISA resource name in"=w831) -> ("error out"=w829:errorcluster, "VISA resource name out"=w830:refnum<visa-resource-name>)  [unwired: 1 out]
          }
          frame #2 {
            # "go back to start"
            n476 = call "Set Stage Position.vi"("Position"=w835, "error in"=w836, "VISA resource name in"=w837) -> ()  [unwired: 3 out]